vi "Core_Chem_User_Interface_v1.4.vi"() -> ()   [LabVIEW 2014]
uses:
  <vilib>/dex/Stream Element Allocation Mode.ctl
  C:/Program Files (x86)/National Instruments/LabVIEW 2014/examples/Data Communication/Network Streams/Simple Network Streams/support/Network Stream Command.ctl
  <vilib>/Platform/TimedLoop/XDataNode/timing_clust.ctl
  <vilib>/Platform/TimedLoop/XDataNode/nitl_modes.ctl
  <vilib>/Platform/TimedLoop/XDataNode/wakeup.ctl
  <vilib>/Utility/tcp.llb/UDP Multicast Read-Only Open.vi
  <vilib>/platform/TimedLoop/XDataNode/XDataNode.xnode
  <vilib>/Platform/TimedLoop/XDataNode/XDNodeRunTimeDep.lvlib
  <vilib>/FTP/NI_FTP.lvlib
panel:
  out "Create folder error out 2":errorcluster
  out "Network to cRIO live status":bool
  out "Create folder error out":errorcluster
  in  "Confirm Flight Number":bool
  out "PRTAFT_UDP_In":string
  out "TWBOZO01":string
  out "CABOZO01":string
  out "TEIOZO01":string
  out "CHTSOO01":string
  out "CHFGGA01":string
  out "AL52CO01":string
  in  "Flight Number":string
  in  "Tab Control":T1(tab)
  out "FGGA preflight Des 17":string="Preflight - Start minimum 2 hours before take-off\n\n1. Ensure no bags/jackets are stowed on seat backs and behind seats in front of core chemistry rack at all times.\n\n2. Remove inlet covers if applicable.\n\n3. Connect Lilliput mini TFT/LCD VGA cable to FGGA VIDEO (back panel) and PS2 Keyboard/Mouse cables to FGGA Connectors (back panel). TFT/LCD and Keyboard kept in Core Chemistry Dell laptop bag. Connect TFT/LCD AC/DC PSU to 6026-8-98 Amphenol (SSP9) and make 230 Vac CB.\n\n4. Ensure all circuit breakers are pushed in, except 230Vac and 28Vdc, UPS switch off (down) and AL5002 CO Plasma Lamp switch off (down), WoW key to normal (horizontal).\n\n5. Wait for ALL network swtiches on the aircraft to be up and running before start-up.\n\n6. Check AboutTime has synchronised laptop clock to aircraft timeservers (Filiberto/Gaston).\n\nClick the PowerUp Tab."
  out "FGGA preflight Des 16":string="PowerUp\n\n1.\tSSP9 forward face\tMake 3 CBs\n\n2.\tPWRDIST \t\tMake 230Vac CB \n                     Switch UPS On \t[UP]\n                     Make 28Vdc CB\n                     Check 28VDC OK Green Light comes on\n\n3.\tCore Chemistry e-Log\nComplete Core Chemistry e-Log in WordPad (Bnnn_CoreChemLog_v2.2), save on Flight Manager's laptop (192.168.101.180/      flt_folders/Bnnn); Fill in header with date, flight number and your name/initials.\n\n4.\tSAMPUMP\t\t\n - Switch WoW override key (vertical) to check pump starts, and MFM flowrate increase (>20 LPM) on the right hand plot. \n - Switch off WoW override\t\t\t\t [NORM, key horizontal]\n\nClick the 2B Ozone tab if operated, otherwise, click the UDP tab.\n\n\n"
  out "MFM":dbl(graph)
  in  "Ambient = OFF\nCabin = ON":bool
  out "FGGA preflight Des 15":string="2B Ozone Preflight\n\n1.\tSelect either Ambient or Cabin Air mode (default should be OFF for Ambient air mode).\n\n2. Check flowrate is greater than 2000 sccm on the right hand plot.\n\nClick the UDP tab."
  out "2B Ozone concentration":dbl(graph)
  out "2B Ozone flow rate":dbl(graph)
  out "2BOzone Event error out":errorcluster
  out "2BOzone command sender error out":errorcluster
  out "FGGA preflight Des 20":string="4. Check derived parameters in DECADES (192.168.101.110 & 192.168.101.108). 574 Ozone TEi49C; 588 CO AL5002; 611 SO2 TEi43i; 903 - 905 FGGA; 910 / 920 Ozone 2B."
  out "FGGA preflight Des 14":string="UDP Preflight\n1. Check all UDP packets are updating.  Unix time increasing by 1 sec (3rd parameter).\n2. Check flight number is correct.\n3. Confirm flight number and check it appears in the UDP packet (6th parameter). "
  in  "name":string="239.1.4.6"
  in  "Port":u16=50001
  out "FGGA":string
  out "CO":string
  out "Ozone":string
  out "Cabin Ozone":string
  out "Ambient Ozone":string
  out "SO2":string
  out "Ozone Zeroing\nTime Remain (sec)":u32
  in  "Ozone Zeroing":bool
  out "TEI49C Sample Flow B":dbl(graph)
  out "TEi49C Concentration":dbl(graph)
  out "TEI49C Sample Flow A":dbl(graph)
  out "FGGA preflight Des 13":string="TEi49C Ozone PRE-FLIGHT - LAST ACTIONS BEFORE SEAT-BELTING DOWN (PRIOR TO ENGINES START)\n\n1. Ozone monitor zeroing\t\t[10 min minimum]\n\n\n2. Check TEi49C zero value and note down value in e-Log. \n"
  out "FGGA preflight Des 12":string="TEi49C Ozone Preflight\n\n1. Check nominal sample flowrate on both channels is ~0.7 LPM."
  out "Ozone Event error out":errorcluster
  out "Ozone command sender error out":errorcluster
  in  "Ozone UDP Time Offset":i32=1
  in  "eV9 Flush User\nset time (sec)":i32=15
  in  "MFC_3 User Set Value":dbl=2.0
  in  "MFC_2 User Set Value":dbl=2.5
  out "SO2 Zeroing (Inflight)\nTime Remain (sec)":u32
  in  "eV6 User set time \n(Inflight) (sec)":i32=120
  in  "eV6 User\nset time (sec)":i32=600
  in  "SO2 Inflight \nZeroing":bool
  out "SO2 Flush\nTime Remain (sec)":u32
  out "TEI43i MFC3 Sample Flow":dbl(graph)
  out "TEi43C / TEi43i Concentration":dbl(graph)
  out "TEI43C Sample Flow":dbl(graph)
  out "TEI43i MFC2 Cal Flow":dbl(graph)
  out "SO2 CAL\nTime Remain (sec)":u32
  out "SO2 Cal Flush\nTime Remain (sec)":u32
  in  "SO2 CAL":bool
  out "FGGA preflight Des 11":string="TEi43 SO2 Inflight Calibration & Zeroing"
  in  "SO2 Zeroing":bool
  out "SO2 Zeroing\nTime Remain (sec)":u32
  out "FGGA preflight Des 10":string="TEi43 SO2 PRE-FLIGHT - LAST ACTIONS BEFORE SEAT-BELTING DOWN (PRIOR TO ENGINES START)\n\n1. SO2 monitors zeroing\t\t[10 min minimum]\n\n\n2. Check TEi43i or TEi43C zero value and note down value in e-Log. "
  in  "SO2 Flush":bool
  out "FGGA preflight Des 9":string="TEi43 SO2 Preflight\n\n1. Check nominal sample flowrate is 2.0 LPM on the right hand plot.\n\nSO2 calibration gas purge - SO2 calibration cylinder locate at bottom of WAS Gas rack.\n\n2. Check quick connect male body is connected to 'chem 1' gas line.\n\n3. Open cylinder valve 1.\n\n4. Set regulator (V2) to deliver at 3 bar.\n\n5. Open regulator valve 3 (anti-clockwise).\n\n6. Close cylinder valve 1.\n\n\n7. Press SO2 flush button, MFC2 cal flow should increase to 2.5 SLPM.\nMonitor MFC2 flow rate to make sure the reading decreases from 2.5 SLPM to 0.0 SLPM.\nCheck pressure content and delivery gauges also reads zero.\nIf pressure content & delivery gauges do NOT read zero, press SO2 flush button again until they do.\n\n8. Quickly open and close cylinder valve 1.\n\n9. Repeat step 7) to 8) three times.\n\n10. Open cylinder valve 1, system is ready. Note down content pressure in elog.\n "
  in  "eV9 flush User\nset time (sec)":i32=60
  in  "eV8 User\nset time (sec)":i32=120
  out "SO2 Event error out":errorcluster
  out "SO2 command sender \nerror out":errorcluster
  in  "SO2 UDP Time Offset":i32=1
  out "Lamp Temperature":dbl(graph)
  out "CO CAL Status":bool
  in  "CO CAL":bool
  out "FGGA preflight Des 8":string="CO Preflight and Inflight Calibrations\nHold down the CAL button for 2 secs then release, CAL status should then lit up.\nInflight calibration performed on 45 minutes interval or more frequently if lamp temperature > 35.5 degC."
  in  "Prepare Gases":bool
  out "FGGA preflight Des 7":string="AL5002 CO Preflight Checks\n\n1.\n\n2. Start CO Vacuum. NB: If there is problem with the software control, use manual override switch [up] on CALDECK front panel\n\n3. CO Checks - charts on the right hand side\n    Lamp Flow Controller ~ 40 ml/min\n    Monochromator Flow Controller ~ 30 ml/min\n    Fluorescence Cell Pressure ~ 7.5 Torr\n\nIf Lamp/Mono flows are low, manual valves (V1 -> V5) may still be shut, or pressure adjusting valves (ALREG1 & 2) have not been set > 2 bar\n\nIf Cell pressure is 10 Torr (max range), check that COPUMP is running and eV7 is opened (CO Vacuum eV7 is ON).\n\n4. Switch Plasma Lamp at the front panel UP\n\nDetector count rate (on 'Raw Signal' or F2 instrument touchscreen) should increase to >=10000 Hz within a minute.  Recycle plasma lamp switch (off/on) if no significant increase in count rate after 10 mins.  CO concentration should increase (100s ppb). \n     \n\n"
  in  "CO Vaccum (eV7)":bool
  out "Raw Signal":dbl(graph)
  out "CO Concentration":dbl(graph)
  out "Fluorescence Cell Pressure":dbl(graph)
  out "Monochromator Flow":dbl(graph)
  out "Lamp Flow Controller":dbl(graph)
  in  "CO UDP Time Offset":i32=1
  out "CO2 Pressure\nDelivery (PSIA)":dbl(slide) scale=0.0..100.0
  out "Std\nContent (barG)":dbl(slide) scale=0.0..220.0
  out "N2\nContent (barG)":dbl(slide) scale=0.0..220.0
  out "CO2\nContent (barG)":dbl(slide) scale=0.0..170.0
  out "CO Event error out":errorcluster
  out "CO command sender error out":errorcluster
  out "CO Zero":T2(array[cluster])
  out "CO Sensitivity":T3(array[cluster])
  out "Ring Down Time RDA & RDB":cluster{dbl, dbl}(graph)
  in  "Line Lock Setting Change":bool
  out "Cell temperature":dbl(graph)
  out "Cell pressure":dbl(graph)
  in  "Manual FGGA Pump":bool
  out "CO2":dbl(graph)
  out "CH4":dbl(graph)
  out "H2O":dbl(graph)
  out "WoW Flag":string="0"
  in  "FGGA pump\nsync to WoW":bool
  out "CH4 Dry":dbl(graph)
  out "CO2 Dry":dbl(graph)
  out "MFC1 Cal Flow":dbl(graph)
  out "Flush Target Tank\nTime Remain (sec)":u32
  out "Flush Low Tank\nTime Remain (sec)":u32
  out "Flush High Tank\nTime Remain (sec)":u32
  in  "Flush Target Tank":bool
  in  "Flush Low Tank":bool
  in  "Flush High Tank":bool
  in  "FGGA Restart":bool
  out "FGGA preflight Des 6":string="FGGA Instrument Controls"
  in  "High Cal":bool
  out "High Cal\nFlush Time Remain (sec)":u32
  out "High Cal\nCal Time Remain (sec)":u32
  in  "Low Cal":bool
  in  "Target Cal":bool
  in  "Span Cal - \nHigh Cal, CO Cal, Low Cal":bool
  out "Low Cal\nFlush Time Remain (sec)":u32
  out "Low Cal\nCal Time Remain (sec)":u32
  out "Target Cal\nFlush Time Remain (sec)":u32
  out "Target Cal\nCal Time Remain (sec)":u32
  in  "MFC_1 User Set Value":dbl=2.0
  out "FGGA preflight Des 5":string="FGGA Inflight Calibrations"
  out "FGGA preflight Des 4":string="FGGA Ground Preflight Checks\n\n1. Switch FGGA pump ON\n\n2. Check cavity pressure ~50 Torr\n\n3. Switch FGGA pump OFF\n\n4. Enable FGGA pump sync to WoW\n\n5.. Check Time Synchronisation\n\n6. Check CO2 & CH4 values\n\nIf CO2 & CH4 values are -1 ppm, follow the \nchange linelock settings procedure.\n\n\n\n\n\nLAST ACTION BEFORE SEAT-BELTING \nDOWN (PRIOR TO ENGINES START)\n\n1. Disconnect Monitor & stow away. Leave Keyboard & Mouse connected. Place keyboard at the bottom\nof the rack.\n\n"
  out "FGGA preflight Des 3":string="FGGA CAL Gas Purge\n\nFor each cylinder in gas stowage, check that,\n\n1. V1 Closed\n    V3 Closed\n    V4 Make sure arrow positioned downwards (i.e. flow points to gas line)\n\n2. V3 Open (turn anti-clockwise)\n\n3. Use the button on the right according to the operating cylinder to flush the line. Monitor the MFC flow rate to make sure the reading decreases from 3 to zero. (ie fully flushed). Pressure content & delivery gauges should also read zero.\n\n4. V3 Close (turn clockwise)\n\n5. V1 Open / Close quickly\n         Check delivery pressure gauge is ~ 40 PSI \n         (Use V2 to increase if necessary)\n\n6. Repeat steps 2) to 5) three times\n\n7. V3 Close (turn clockwise)\n\n8. V1 Open, check V2 ~ 40 PSIG\n\n9. V3 Open - System is ready"
  out "FGGA command sender error out":errorcluster
  out "FGGA Event Error out":errorcluster
  in  "FGGA UDP Time Offset":i32=1
  in  "FGGA Shutdown":bool
  in  "Postflight Procedures":bool
  in  "cRIO File IO Stop\n(USB Flash Drive Unmount)":bool
  in  "FTP ASCII Files to Local":bool
  in  "Transfer FGGA Files":bool
  out "FGGA preflight Des 18":string="Postflight\n\n1. Press the cRIO File IO Stop to stop ASCII file recording\nNote: ASCII file recording will start again once a new  flight number is confirmed.\n\n2. Press the FTP ASCII File to Local button to transfer ASCII files to flight folder.\n\n\n3. Press the Transfer FGGA Files button to transfer FGGA files to flight folder. \n\n4. Shutdown FGGA.\n\n\n5. View Postflight Procedures."
  out "File List":string[](array[string])
  out "FGGA File Transfer Error out":errorcluster
  out "Move to FM Error out":errorcluster
  out "USB Disk Space Used %":dbl(slide) scale=0.0..100.0
  out "PTP Sync":bool
  out "CPU Total %":dbl(graph)
  out "PRTAFT_DLU":string
  out "FGGA preflight Des 19":string="This tab controls ONLY for advanced operators."
  in  "Inst_alm_thresh":i32=220
  in  "3hr_alm_thresh":i32=80
  in  "Simulate Inst Conc":i32
  in  "Simulate 3hr Average Conc":dbl
  in  "Simulate 2B Conc":bool
  in  "Ozone eV6":bool
  in  "Simulate Conc":bool
  in  "8hr TWA Limit":i32=490
  in  "10mins STEL Limit":i32=700
  in  "SO2 Slope":dbl=1.0
  in  "SO2 Offset":dbl
  in  "Simulate TWA Conc":dbl
  in  "Simulate STEL Conc":dbl
  in  "MFC_3\nSLPM Value":dbl=2.0
  in  "MFC_2\nSLPM Value":dbl
  in  "SO2 eV6":bool
  in  "eV8":bool
  in  "eV9":bool
  in  "eV4":bool
  in  "eV3":bool
  in  "MFC_1\nSLPM Value":dbl
  in  "eV2":bool
  in  "eV1":bool
  # "Unix time"
  # "Flight Number"
  # "Unix time"
  # "Unix time"
  # "Unix time"
  # "Unix time"
  # "concentration\npmt_volt\nlamp_volt\nlamp_intens\ninternal_temper\nreact_temper\nreact_press\nflow\nflags\nten_min_so2\neight_hr_so2\nten_min_so2_alm\neight_hr_so2_alm\nMFC_2absolute_pres\nMFC_2temperature\nMFC_2volumetic_flow\nMFC_2mass_flow\nMFC_2set_point\nMFC_3_absolute_pres\nMFC_3_temperature\nMFC_3volumetic_flow\nMFC_3mass_flow\nMFC_3set_point\nV6\nV8\nV9\nMFC2_Set_Value\nMFC3_Set_Value"
  # "Flight Number"
  # "Flight Number"
  # "Flight Number"
  # "Flight Number"
  # "conc\ntemp\npress\nflow\nthreehr_oz\nInst_alarm\nthreehr_alarm"
  # "ch4\nco2\nh2o\npress_torr\ntemp_c\nfit_flag\nrda_usec\nrdb_usec\nch4_dry\nco2_dry\nMFC_1_absolute_pres\nMFC_1_temperature\nMFC_1volumetic_flow\nMFC_1mass_flow\nMFC_1set_point\nV1\nV2\nV3\nV4\nrestart_FGGA\nFGGA_Pump\nCAL_MFC_1Set_Value"
  # "conc\ntemp\npress\nflow"
  # "conc\nbenchtemp\npress\ncellAint\ncellBint\nFlowA\nFlowB\nlamptemp\nflag\nV6"
  # "conc\ncounts\nsens\nzero\nlampflow\nlamptemp\nmonoflow\nmonotemp\nmonopress\ncellpress\ncalpress\ntemppmt\ncalconc\nerr\ncal_counter\nerr_counter\nCO_vacuum_status\nIn_Cal\nALEG1_press_delivery\nALREG1_press_content\nALREG2_press_content\nALREG3_press_content"
  # "TEi43c"
  # "TEi43i"
  # "V3"
  # "V2"
  # "V1"
  # "SO2 CAL SETTINGS"
  # "FGGA"
  # "2B Ozone"
  # "TEi49C  - Ozone"
  # "TEi43 - SO2"
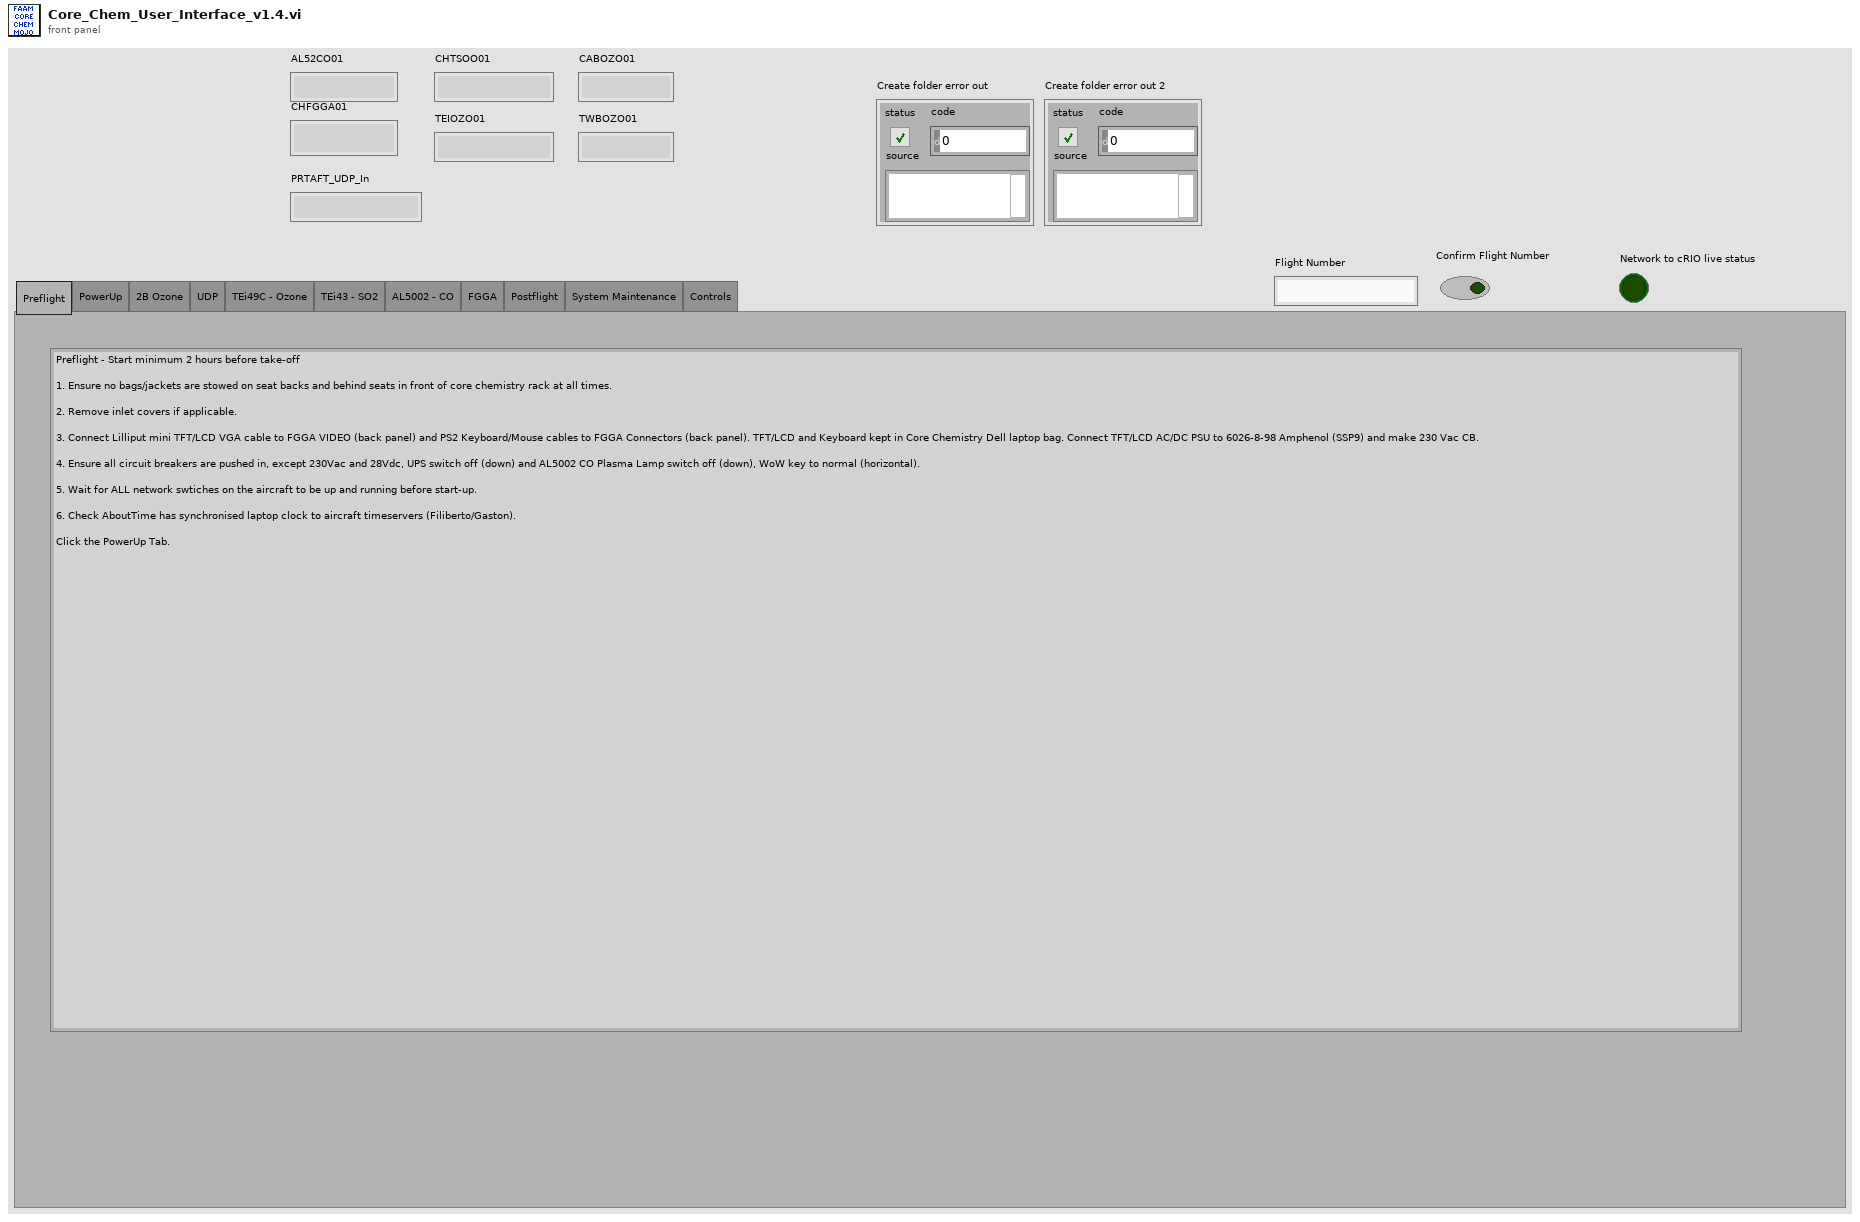
[diagram p1: front panel]
types:
  T1 = enum32{"Preflight", "PowerUp", "2B Ozone", "UDP", "TEi49C - Ozone", "TEi43 - SO2", "AL5002 - CO", "FGGA", "Postflight", "System Maintenance", "Controls"}
  T2 = cluster{"time stamp":timestamp, "CO Offset":dbl}[]
  T3 = cluster{"time stamp":timestamp, "CO Sensitivity":dbl}[]
  T4 = typedef "Network Stream Command.ctl" = cluster{"Message":string, "Message Data":variant}
  T5 = typedef "Stream Element Allocation Mode.ctl" = u32
  T6 = typedef "XDNodeRunTimeDep.lvlib/timing_clust.ctl" = cluster{"Expected End [f-1]":u64, "Actual End [f-1]":u64, "Finished Late? [f-1]":bool, "Expected End [i-1]":u64, "Actual End [i-1]":u64, "Finished Late? [i-1]":bool, "Expected Start [i]":u64, "Actual Start [i]":u64, "Expected Start [f]":u64, "Actual Start [f]":u64, "Source Name":string, "Structure Name":string, "Period":i64, "Deadline":i64, "Offset":i64, "Start":i64, "Priority":i32, "Timeout":i32, "Mode":T7, "Wakeup Reason":T8, "Error":errorcluster, "Source Type":string, "Secondary Source Type":string, "Global End Time":u64, "Global Start Time":u64, "Frame Duration":u64, "Iteration Duration":u64, "Assigned CPU":i32, "I/O Scan Engine Mode":u32}
  T7 = typedef "XDNodeRunTimeDep.lvlib/nitl_modes.ctl" = enum32{"No Change", "Process missed periods, maintain original phase", "Discard missed periods, maintain original phase", "Process missed periods, ignore original phase", "Discard missed periods, ignore original phase"}
  T8 = typedef "XDNodeRunTimeDep.lvlib/wakeup.ctl" = enum32{"Normal", "Aborted", "Asynchronous wakeup", "Timing source error", "Timed loop error", "Timeout"}
  T9 = typedef "NI_FTP.lvlib/FTP Session.ctl" = refnum<k5>
  T10 = typedef "NI_FTP.lvlib/FTP File Info.ctl" = cluster{"type":enum16{"unknown", "file", "dir", "link"}, "permissions":string, "owner":string, "group":string, "size":i32, "date":string, "name":string, "link name":string}
  T11 = cluster{"Message":string, "Message 2":string, "Message 3":string}
  T12 = cluster{"Message":string, "Message 2":string, "Message 3":string, "Message 4":string}
  T13 = cluster{"Message":string, "Message 3":string, "Message 4":string}
diagram:
  w4 = "XXXX"
  w7 = 0
  w8 = 0.0
  w14 = T4 {"Message"="", "Message Data"=variant} ("Message Cluster")
  w20 = T5 0 items=["allocate as needed", "pre-allocate"] ("element allocation mode")
  w26 = T4 {"Message"="", "Message Data"=variant} ("Message Cluster")
  w32 = T5 0 items=["allocate as needed", "pre-allocate"] ("element allocation mode")
  w37 = T4 {"Message"="", "Message Data"=variant} ("Message Cluster")
  w43 = T5 0 items=["allocate as needed", "pre-allocate"] ("element allocation mode")
  w53 = T5 0 items=["allocate as needed", "pre-allocate"] ("element allocation mode")
  w55 = T4 {"Message"="", "Message Data"=variant} ("Message Cluster")
  w62 = T5 0 items=["allocate as needed", "pre-allocate"] ("element allocation mode")
  w64 = T4 {"Message"="", "Message Data"=variant} ("Message Cluster")
  n1 = local write "cRIO File IO Stop\n(USB Flash Drive Unmount)"(FALSE ("Stop File Write")) -> ()
  n2 = local write "Flight Number"(w4) -> ()
  n3 = while {
    shift-right: [w68] -> _
    shift-left: w4 -> [w67]
    stop <- FALSE stop-if-true
    n4 = Not Equal?(x=w67, y="Flight Number") -> (x != y?=w70:bool)
    n5 = case shown="True" w70 {
      tunnel: [w73 w74] -> w68
      tunnel: "Flight Number" -> [_ w74]
      tunnel: w67 -> [w73 _]
      frame False {
      }
      frame True {
        n6 = One Button Dialog(message="Flight Number changed,\nPress flight number button to confirm") -> ()  [unwired: 1 in, 1 out]
      }
    }
    n7 = Wait (ms)(milliseconds to wait=u32 1000) -> ()  [unwired: 1 out]
  }
  n8 = while {
    stop <- FALSE stop-if-true
    # "UDP Read"
    n9 = String To IP(1:"name") -> (0:w81:u32)
    n10 = call-poly <vilib>:"UDP Multicast Open.vi"("multicast addr"=w81, "port"="Port") -> ("error out"=w79:errorcluster, "connection ID"=w78:refnum<k16>)  [unwired: 7 in, 1 out]
    n11 = Wait (ms)(milliseconds to wait=u32 1000) -> ()  [unwired: 1 out]
    n12 = case shown="No Error" w79 {
      selector: w79 -> [w85 _]
      tunnel: w78 -> [w84 _]
      frame No Error {
        w83 = ""
        n13 = while {
          tunnel: w85 -> [w131]
          tunnel: w84 -> [w130]
          shift-right: [w126] -> _
          shift-left: w83 -> [w127]
          shift-right: [w117] -> _
          shift-left: w83 -> [w119]
          shift-right: [w111] -> _
          shift-left: w83 -> [w113]
          shift-right: [w105] -> _
          shift-left: w83 -> [w106]
          shift-right: [w99] -> _
          shift-left: w83 -> [w100]
          shift-right: [w93] -> _
          shift-left: w83 -> [w94]
          shift-right: [w87] -> _
          shift-left: w83 -> [w88]
          stop <- w129 stop-if-true
          n14 = UDP Read(connection ID=w130, 8:w131) -> (data out=w86:string, error out=w129:errorcluster)  [unwired: 2 in, 3 out]
          n15 = Match Pattern(string=w86, regular expression="$TEIOZO01,") -> (match substring=w125:string, after substring=w124:string)  [unwired: 1 in, 2 out]
          n16 = Match Pattern(string=w86, regular expression="$TWBOZO01,") -> (match substring=w103:string, after substring=w102:string)  [unwired: 1 in, 2 out]
          n17 = Match Pattern(string=w86, regular expression="$CABOZO01,") -> (match substring=w109:string, after substring=w108:string)  [unwired: 1 in, 2 out]
          n18 = Match Pattern(string=w86, regular expression="$CHTSOO01,") -> (match substring=w97:string, after substring=w96:string)  [unwired: 1 in, 2 out]
          n19 = Match Pattern(string=w86, regular expression="$CHFGGA01,") -> (match substring=w121:string, after substring=w120:string)  [unwired: 1 in, 2 out]
          n20 = Match Pattern(string=w86, regular expression="$AL52CO01,") -> (match substring=w115:string, after substring=w114:string)  [unwired: 1 in, 2 out]
          n21 = Match Pattern(string=w86, regular expression="$PRTAFT01,") -> (match substring=w92:string, after substring=w91:string)  [unwired: 1 in, 2 out]
          n22 = Concatenate Strings(w125, w124) -> (w123:string)
          n23 = Concatenate Strings(w103, w102) -> (w101:string)
          n24 = Concatenate Strings(w109, w108) -> (w107:string)
          n25 = Concatenate Strings(w97, w96) -> (w95:string)
          n26 = Concatenate Strings(w121, w120) -> (w118:string)
          n27 = Concatenate Strings(w115, w114) -> (w112:string)
          n28 = Concatenate Strings(w92, w91) -> (w89:string)
          n29 = Replace Substring(4:w101, 5:w100) -> (1:w99:string)  [unwired: 2 in, 1 out]
          "TWBOZO01" <- w99
          n30 = Replace Substring(4:w123, 5:w127) -> (1:w126:string)  [unwired: 2 in, 1 out]
          "TEIOZO01" <- w126
          n31 = Replace Substring(4:w107, 5:w106) -> (1:w105:string)  [unwired: 2 in, 1 out]
          "CABOZO01" <- w105
          n32 = Replace Substring(4:w95, 5:w94) -> (1:w93:string)  [unwired: 2 in, 1 out]
          "CHTSOO01" <- w93
          n33 = Replace Substring(4:w112, 5:w113) -> (1:w111:string)  [unwired: 2 in, 1 out]
          "AL52CO01" <- w111
          n34 = Replace Substring(4:w118, 5:w119) -> (1:w117:string)  [unwired: 2 in, 1 out]
          "CHFGGA01" <- w117
          n35 = Replace Substring(4:w89, 5:w88) -> (1:w87:string)  [unwired: 2 in, 1 out]
          "PRTAFT_UDP_In" <- w87
        }
      }
      frame Error {
      }
    }
  }
  n36 = Obtain Queue(name (unnamed)="CO_Command", element data type=w64) -> (queue out=w13:refnum<queue>, error out=w58:errorcluster)  [unwired: 3 in, 1 out]
  n37 = Create Network Stream Writer Endpoint(6:w62, 7:10 ("writer buffer size"), 9:w64, 10:"//192.168.101.17/command/reader/CO" ("reader url"), 11:"/command/writer/CO" ("writer name")) -> (0:w61:errorcluster, 3:w60:refnum<k21>)  [unwired: 2 in]
  n38 = while {
    tunnel: w13 -> [w135]
    tunnel: w58 -> [w134]
    tunnel: [w132] -> _
    stop <- FALSE stop-if-true
    # "CO UI Event Handler Loop"
    n39 = event shown="[4] \"Confirm Flight Number\": Value Change" {
      selector: _ -> [_ _ _ _ _]
      dyn-events: _ -> [_ _ _ _ _]
      timeout: _ -> [_ _ _ _ _]
      tunnel: w135 -> [w142 w149 w153 w160 w168]
      tunnel: w134 -> [w141 w148 w152 w159 w167]
      tunnel: [w136 w143 w151 w158 w166] -> w132
      event "CO CAL": Value Change {
        n40 = event-data() -> ("NewVal"=w139:bool)  [unwired: 1 in]
        n41 = Bundle(cluster=T4 {"Message"="", "Message Data"=variant} ("Message Cluster"), "Message"="CO CAL", "Message Data"=w139) -> (w137:T4)
        n42 = Enqueue Element(queue=w142, element=w137, error in (no error)=w141) -> (error out=w136:errorcluster)  [unwired: 1 in, 2 out]
      }
      event "CO UDP Time Offset": Value Change {
        n43 = event-data() -> ("NewVal"=w146:i32)  [unwired: 1 in]
        n44 = Bundle(cluster=T4 {"Message"="", "Message Data"=variant} ("Message Cluster"), "Message"="UDP Time Offset", "Message Data"=w146) -> (w144:T4)
        n45 = Enqueue Element(queue=w149, element=w144, error in (no error)=w148) -> (error out=w143:errorcluster)  [unwired: 1 in, 2 out]
      }
      event "CO Vaccum (eV7)": Value Change {
        n46 = event-data() -> ("NewVal"=w150:bool)  [unwired: 1 in]
        n47 = Bundle(cluster=T4 {"Message"="", "Message Data"=variant} ("Message Cluster"), "Message"="CO Vacuum", "Message Data"=w150) -> (w154:T4)
        n48 = Enqueue Element(queue=w153, element=w154, error in (no error)=w152) -> (error out=w151:errorcluster)  [unwired: 1 in, 2 out]
      }
      event "cRIO File IO Stop\n(USB Flash Drive Unmount)": Value Change {
        n49 = event-data() -> ("NewVal"=w157:bool)  [unwired: 1 in]
        n50 = Bundle(cluster=T4 {"Message"="", "Message Data"=variant} ("Message Cluster"), "Message"="Stop File Write", "Message Data"=w157) -> (w161:T4)
        n51 = Enqueue Element(queue=w160, element=w161, error in (no error)=w159) -> (error out=w158:errorcluster)  [unwired: 1 in, 2 out]
      }
      event "Confirm Flight Number": Value Change {
        n52 = event-data() -> ()  [unwired: 1 in, 1 out]
        n53 = flat-sequence {
          tunnel: w167 -> [w170]
          tunnel: w168 -> [w171]
          tunnel: [w171] -> w165
          tunnel: [w170] -> w164
          tunnel: [w173] -> w166
          tunnel: w165 -> [w175]
          tunnel: w164 -> [w174]
          frame #0 {
            n54 = local write "cRIO File IO Stop\n(USB Flash Drive Unmount)"(FALSE ("cRIO File IO Stop\n(USB Flash Drive Unmount)")) -> ()
          }
          frame #1 {
            n55 = local read "Flight Number"() -> (w172:string)
            n56 = Bundle(cluster=T4 {"Message"="", "Message Data"=variant} ("Message Cluster"), "Message"="Flight Number", "Message Data"=w172) -> (w176:T4)
            n57 = Enqueue Element(queue=w175, element=w176, error in (no error)=w174) -> (error out=w173:errorcluster)  [unwired: 1 in, 2 out]
          }
        }
      }
    }
    "CO Event error out" <- w132
  }
  n58 = while {
    tunnel: w13 -> [w186]
    shift-right: [w181] -> _
    shift-left: w60 -> [w183]
    shift-right: [w179] -> w49
    shift-left: w61 -> [w185]
    tunnel: w58 -> [w180]
    stop <- w179 stop-if-true
    # "CO UI Command Sender"
    n59 = Dequeue Element(queue=w186, error in (no error)=w180) -> (element=w182:T4)  [unwired: 1 in, 3 out]
    n60 = Unbundle By Name(w182) -> ("Message"=w184:string)
    n61 = case shown="\"UDP Time Offset\"" w184 {
      tunnel: w185 -> [w187 w191 w198 w205 w212 w219]
      tunnel: w183 -> [w188 w194 w201 w208 w215 w222]
      tunnel: w182 -> [_ w193 w200 w207 w214 w221]
      tunnel: [w187 w190 w197 w204 w211 w218] -> w179
      tunnel: [w188 w189 w196 w203 w210 w217] -> w181
      frame "False", Default {
      }
      frame "CO CAL" {
        n62 = shared-variable-write(w194, w191, w193) -> (w192:refnum<k21>, w195:errorcluster)  [unwired: 1 in, 1 out]
        n63 = Flush Stream(8:w195, 11:w192) -> (0:w190:errorcluster, 3:w189:refnum<k21>)  [unwired: 2 in, 1 out]
      }
      frame "UDP Time Offset" {
        n64 = shared-variable-write(w201, w198, w200) -> (w199:refnum<k21>, w202:errorcluster)  [unwired: 1 in, 1 out]
        n65 = Flush Stream(8:w202, 11:w199) -> (0:w197:errorcluster, 3:w196:refnum<k21>)  [unwired: 2 in, 1 out]
      }
      frame "Stop File Write" {
        n66 = shared-variable-write(w208, w205, w207) -> (w206:refnum<k21>, w209:errorcluster)  [unwired: 1 in, 1 out]
        n67 = Flush Stream(8:w209, 11:w206) -> (0:w204:errorcluster, 3:w203:refnum<k21>)  [unwired: 2 in, 1 out]
      }
      frame "Flight Number" {
        n68 = shared-variable-write(w215, w212, w214) -> (w213:refnum<k21>, w216:errorcluster)  [unwired: 1 in, 1 out]
        n69 = Flush Stream(8:w216, 11:w213) -> (0:w211:errorcluster, 3:w210:refnum<k21>)  [unwired: 2 in, 1 out]
      }
      frame "CO Vacuum" {
        n70 = shared-variable-write(w222, w219, w221) -> (w220:refnum<k21>, w223:errorcluster)  [unwired: 1 in, 1 out]
        n71 = Flush Stream(8:w223, 11:w220) -> (0:w218:errorcluster, 3:w217:refnum<k21>)  [unwired: 2 in, 1 out]
      }
    }
  }
  "CO command sender error out" <- w49
  n72 = node-c288() -> (w12:T6)  [unwired: 4 in]
  n73 = Initialize Array(cluster{"time stamp":timestamp, "Y":dbl} {"time stamp"=timestamp(0 s since 1904-01-01), "Y"=0.0}, 30 ("dimension size")) -> (w9:cluster{"time stamp":timestamp, "Y":dbl}[])
  n74 = timed-loop {
    timing: w12 -> [_]
    timing-out: [_] -> w11
    stop <- _ stop-if-true
    # "PC Tasks"
    n75 = node-c288() -> ()  [unwired: 1 in, 1 out]
    n76 = event shown="[0] \"FTP ASCII Files to Local\": Value Change" {
      selector: _ -> [_ _ _ _]
      dyn-events: _ -> [_ _ _ _]
      timeout: _ -> [_ _ _ _]
      event "FTP ASCII Files to Local": Value Change {
        n77 = event-data() -> ()  [unwired: 1 in, 1 out]
        n78 = flat-sequence {
          tunnel: [w232] -> w226
          tunnel: [w244] -> w231
          tunnel: [w243] -> w229
          tunnel: [w242] -> w227
          tunnel: w226 -> [w242]
          tunnel: w231 -> [w302]
          tunnel: [w302] -> w230
          tunnel: w229 -> [w298]
          tunnel: [w297] -> w228
          tunnel: w227 -> [w297]
          tunnel: w230 -> [w308]
          tunnel: w228 -> [w303]
          frame #0 {
            n79 = local read "Flight Number"() -> (w234:string)
            n80 = Concatenate Strings("Confirm Flight Number" ("message"), "\n", w234) -> (w238:string)
            n81 = Two Button Dialog(message=w238, 1:"No" ("F button name (\"Cancel\")"), 2:"Yes" ("T button name (\"OK\")")) -> (T button?=w235:bool)
            n82 = case shown="False" w235 {
              tunnel: w234 -> [_ w241]
              tunnel: [w240 w241] -> w232
              frame False {
                n83 = call "Prompt User for Flight Number2"() -> ("Flight Number BXXX"=w240:string)  [unwired: 17 in, 2 out]
              }
              frame True {
              }
            }
          }
          frame #1 {
            n84 = Get Date/Time In Seconds() -> (seconds since 1Jan1904=w248:timestamp)
            n85 = Format Date/Time String(time format string (%c)="%Y%m%d", seconds (now)=w248) -> (date/time string=w246:string)  [unwired: 1 in]
            n86 = call <vilib>:"FTP Open Session.vi"("address"="192.168.101.17") -> ("error out"=w263:errorcluster, "ftp session"=w264:T9)  [unwired: 7 in, 2 out]
            n87 = Concatenate Strings("Use Today's Date" ("message"), "\r", w246) -> (w252:string)
            n88 = call <vilib>:"FTP Logon.vi"("error in (no error)"=w263, "password"="", "user"="anonymous", "ftp session"=w264) -> ("error out"=w260:errorcluster, "ftp session out"=w259:T9)  [unwired: 4 in, 2 out]
            n89 = Two Button Dialog(message=w252, 1:"No" ("F button name (\"Cancel\")"), 2:"Yes" ("T button name (\"OK\")")) -> (T button?=w249:bool)
            n90 = case shown="False" w249 {
              tunnel: [w267 w268] -> w243
              tunnel: w246 -> [_ w268]
              frame False {
                n91 = call "Prompt User for Date"() -> ("Date"=w267:string)  [unwired: 17 in, 2 out]
              }
              frame True {
              }
            }
            n92 = call <vilib>:"FTP Directory Listing.vi"("error in (no error)"=w260, "directory path"="/U:/data", "ftp session"=w259) -> ("dir list"=w258:T10[])  [unwired: 4 in, 4 out]
            n93 = for {
              tunnel: w258 -> [w288] mode=indexing
              tunnel: [w287] -> w255 mode=indexing
              tunnel: w243 -> [w286]
              # "Extract File Name According to the Date"
              n94 = Unbundle By Name(w288) -> ("name"=w294:string, "name"=w293:string)
              n95 = Match Pattern(string=w293, regular expression="_[0-9]+") -> (match substring=w291:string)  [unwired: 1 in, 3 out]
              n96 = String Subset(string=w291, offset (0)=1) -> (substring=w289:string)  [unwired: 1 in]
              n97 = Equal?(x=w289, y=w286) -> (x = y?=w295:bool)
              n98 = case shown="False" w295 {
                tunnel: w294 -> [_ w296]
                tunnel: [_ w296] -> w287
                frame False {
                }
                frame True {
                }
              }
            }
            n99 = Array Size(array=w255) -> (size(s)=w257:i32)
            n100 = for {
              N: w257 -> [_]
              shift-right: [w275] -> w245
              shift-left: w255 -> [w276]
              shift-right: [w273] -> _
              shift-left: 0 -> [w274]
              # "Remove Empty Array"
              n101 = Index Array(array=w276, index=w274) -> (element=w278:string)
              n102 = Equal?(x=w278, y="") -> (x = y?=w277:bool)
              n103 = case shown="True" w277 {
                tunnel: w276 -> [w282 w285]
                tunnel: w274 -> [w281 w283]
                tunnel: [w282 w284] -> w275
                tunnel: [w280 w283] -> w273
                frame False {
                  n104 = Increment(x=w281) -> (x+1=w280:i32)
                }
                frame True {
                  n105 = Delete From Array(array=w285, index=w283) -> (array with subset deleted=w284:string[])  [unwired: 1 in, 1 out]
                }
              }
            }
            "File List" <- w245
            n106 = for {
              tunnel: w245 -> [w271] mode=indexing
              tunnel: [w269] -> w244 mode=indexing
              # "Specify destination path for each file"
              n107 = Concatenate Strings("C:\\temp\\", w271) -> (w270:string)
              n108 = String To Path(string=w270) -> (path=w269:path)
            }
          }
          frame #2 {
            # "FTP a list of files"
            n109 = call <vilib>:"System Exec.vi"("wait until completion? (T)"=TRUE, "working directory"=path "C:/temp", "standard input"=w298, "command line"="C:\\temp\\transfer_ascii_files.bat") -> ()  [unwired: 4 in, 4 out]
          }
          frame #3 {
            # "Move file from local PC to Flight Folder"
            n110 = Build Path(base path=path "\\\\192.168.101.180\\flt_folders" ("path"), name or relative path=w303) -> (appended path=w310:path)
            n111 = Concatenate Strings(w303, "_" ("string"), "corechem" ("string")) -> (w309:string)
            n112 = Build Path(base path=w310, name or relative path=w309) -> (appended path=w305:path)
            n113 = Create Folder(path (use dialog)=w305) -> (created path=w304:path, error out=→"Create folder error out 2":errorcluster)  [unwired: 2 in, 1 out]
            n114 = for {
              tunnel: w304 -> [w317]
              tunnel: [w316] -> w307
              tunnel: w308 -> [w314] mode=indexing
              n115 = Copy(9:TRUE ("overwrite (F)"), 10:w317, 11:w314) -> (0:w316:errorcluster)  [unwired: 2 in, 2 out]
            }
            "Move to FM Error out" <- w307
          }
          frame #4 {
            n116 = local write "FTP ASCII Files to Local"(FALSE ("FTP Files to Local")) -> ()
          }
        }
      }
      event "Transfer FGGA Files": Value Change {
        n117 = event-data() -> ()  [unwired: 1 in, 6 out]
        n118 = flat-sequence {
          tunnel: [w323] -> w322
          tunnel: w322 -> [w335]
          tunnel: [w335] -> w321
          tunnel: [w334] -> w320
          tunnel: [w333] -> w319
          tunnel: w321 -> [w345]
          tunnel: w320 -> [w344]
          tunnel: w319 -> [w346]
          frame #0 {
            n119 = local read "Flight Number"() -> (w324:string)
            n120 = Concatenate Strings("Confirm Flight Number" ("message"), "\n", w324) -> (w326:string)
            n121 = Two Button Dialog(message=w326, 1:"No" ("F button name (\"Cancel\")"), 2:"Yes" ("T button name (\"OK\")")) -> (T button?=w330:bool)
            n122 = case shown="False" w330 {
              tunnel: w324 -> [_ w332]
              tunnel: [w331 w332] -> w323
              frame False {
                n123 = call "Prompt User for Flight Number"() -> ("Flight Number BXXX"=w331:string)  [unwired: 17 in, 2 out]
              }
              frame True {
              }
            }
          }
          frame #1 {
            n124 = Two Button Dialog(message="Get FGGA Files\nof Today's Date?", 1:"No" ("F button name (\"Cancel\")"), 2:"Yes" ("T button name (\"OK\")")) -> (T button?=w339:bool)
            n125 = case shown="False" w339 {
              selector: w339 -> [w341 w342]
              tunnel: [w341 w342] -> w333
              tunnel: [w340 _] -> w334
              frame False {
                n126 = call "Prompt User for Date"() -> ("Date"=w340:string)  [unwired: 17 in, 2 out]
              }
              frame True {
              }
            }
          }
          frame #2 {
            n127 = Build Path(base path=path "\\\\192.168.101.180\\flt_folders" ("path"), name or relative path=w345) -> (appended path=w350:path)
            n128 = Concatenate Strings(w345, "_" ("string"), "corechem" ("string")) -> (w349:string)
            n129 = Build Path(base path=w350, name or relative path=w349) -> (appended path=w343:path)
            n130 = Create Folder(path (use dialog)=w343) -> (error out=→"Create folder error out":errorcluster)  [unwired: 2 in, 2 out]
            n131 = call "labSSH_FGGA_Files_Transfer.vi"("Flight_num"=w345, "Get current?"=w346, "Date"=w344, "Flight Folder Path"=w343) -> ("error IO"=→"FGGA File Transfer Error out":errorcluster)  [unwired: 11 in]
          }
          frame #3 {
            n132 = local write "Transfer FGGA Files"(FALSE) -> ()
          }
        }
      }
      event "FGGA Restart": Value Change {
        n133 = event-data() -> ()  [unwired: 1 in, 6 out]
        n134 = flat-sequence {
          frame #0 {
            n135 = Two Button Dialog(message="FGGA will be restarted,\nARE YOU SURE?") -> (T button?=w356:bool)  [unwired: 2 in]
            n136 = case shown="True" w356 {
              frame False {
              }
              frame True {
                n137 = call "labSSH_Commands.vi"("Data"="reboot") -> ()  [unwired: 14 in, 1 out]
              }
            }
          }
          frame #1 {
            n138 = local write "FGGA Restart"(FALSE ("FGGA Restart")) -> ()
          }
        }
      }
      event "FGGA Shutdown": Value Change {
        n139 = event-data() -> ()  [unwired: 1 in, 6 out]
        n140 = flat-sequence {
          frame #0 {
            n141 = Two Button Dialog(message="FGGA will be shutdown,\nARE YOU SURE?") -> (T button?=w360:bool)  [unwired: 2 in]
            n142 = case shown="True" w360 {
              frame False {
              }
              frame True {
                n143 = call "labSSH_Commands.vi"("Data"="halt") -> ()  [unwired: 14 in, 1 out]
              }
            }
          }
          frame #1 {
            n144 = local write "FGGA Shutdown"(FALSE ("FGGA Restart")) -> ()
          }
        }
      }
    }
    n145 = node-c288() -> ()  [unwired: 1 in, 1 out]
  }
  n146 = while {
    shift-right: [w459] -> _
    shift-left: w8 -> [w457]
    shift-right: [w461] -> _
    shift-left: w7 -> [w462]
    shift-right: [w460] -> _
    shift-left: w9 -> [w464]
    shift-right: [w453] -> _
    shift-left: w9 -> [w455]
    shift-right: [w450] -> _
    shift-left: w8 -> [w449]
    shift-right: [w452] -> _
    shift-left: w7 -> [w454]
    shift-right: [w446] -> _
    shift-left: FALSE -> [w447]
    stop <- FALSE stop-if-true
    w393 = ""
    w388 = "%s" ("format string")
    w583 = "%s" ("format string")
    w588 = "%s" ("format string")
    w593 = "%s" ("format string")
    w599 = "%s" ("format string")
    w605 = "%s" ("format string")
    w609 = "%s" ("format string")
    # "UDP Data Processing"
    n147 = local read "CHFGGA01"() -> (w612:string)
    n148 = local read "TWBOZO01"() -> (w587:string)
    n149 = local read "AL52CO01"() -> (w604:string)
    n150 = local read "CABOZO01"() -> (w592:string)
    n151 = local read "TEIOZO01"() -> (w598:string)
    n152 = local read "CHTSOO01"() -> (w582:string)
    n153 = local read "PRTAFT_UDP_In"() -> (w386:string)
    n154 = local read "Ambient = OFF\nCabin = ON"() -> (w486:bool)
    n155 = Spreadsheet String To Array(delimiter (Tab)=",", format string=w609, spreadsheet string=w612, array type (2D Dbl)=string[] []) -> (array=w559:string[])
    n156 = Spreadsheet String To Array(delimiter (Tab)=",", format string=w605, spreadsheet string=w604, array type (2D Dbl)=string[] []) -> (array=w580:string[])
    n157 = Spreadsheet String To Array(delimiter (Tab)=",", format string=w593, spreadsheet string=w592, array type (2D Dbl)=string[] []) -> (array=w483:string[])
    n158 = Spreadsheet String To Array(delimiter (Tab)=",", format string=w599, spreadsheet string=w598, array type (2D Dbl)=string[] []) -> (array=w557:string[])
    n159 = Spreadsheet String To Array(delimiter (Tab)=",", format string=w588, spreadsheet string=w587, array type (2D Dbl)=string[] []) -> (array=w482:string[])
    n160 = Spreadsheet String To Array(delimiter (Tab)=",", format string=w583, spreadsheet string=w582, array type (2D Dbl)=string[] []) -> (array=w555:string[])
    n161 = Array To Spreadsheet String(delimiter (Tab)="\r", array=w559, 3:w609) -> (spreadsheet string=→"FGGA":string)
    n162 = Array To Spreadsheet String(delimiter (Tab)="\r", array=w580, 3:w605) -> (spreadsheet string=→"CO":string)
    n163 = Array To Spreadsheet String(delimiter (Tab)="\r", array=w483, 3:w593) -> (spreadsheet string=→"Cabin Ozone":string)
    n164 = Array To Spreadsheet String(delimiter (Tab)="\r", array=w557, 3:w599) -> (spreadsheet string=→"Ozone":string)
    n165 = Spreadsheet String To Array(delimiter (Tab)=",", format string=w388, spreadsheet string=w386, array type (2D Dbl)=string[] []) -> (array=w387:string[])
    n166 = Array To Spreadsheet String(delimiter (Tab)="\r", array=w482, 3:w588) -> (spreadsheet string=→"Ambient Ozone":string)
    n167 = Array To Spreadsheet String(delimiter (Tab)="\r", array=w555, 3:w583) -> (spreadsheet string=→"SO2":string)
    n168 = Array To Spreadsheet String(delimiter (Tab)="\r", array=w387, 3:w388) -> (spreadsheet string=→"PRTAFT_DLU":string)
    n169 = Index Array(array=w387, index #1=5 ("index"), index #2=19 ("index")) -> (element #1=w391:string, element #2=w389:string)
    n170 = Select(t=w483, s=w486, f=w482) -> (s? t:f=w481:string[])
    n171 = Not Equal?(x=w391, y=w393) -> (x != y?=w392:bool)
    n172 = Not Equal?(x=w389, y=w393) -> (x != y?=w390:bool)
    n173 = Index Array(array=w555, index #1=6 ("index"), index #2=4 ("index"), index #3=3 ("index"), index #4=7 ("index"), index #5=8 ("index"), index #6=15 ("index"), index #7=24 ("index"), index #8=29 ("index")) -> (element #1=w472:string, element #2=w538:string, element #3=w533:string, element #4=w526:string, element #5=w502:string, element #6=w501:string, element #7=w411:string, element #8=w410:string)
    n174 = Index Array(array=w481, index #1=8 ("index"), index #2=11 ("index")) -> (element #1=w475:string, element #2=w476:string)
    n175 = Index Array(array=w557, index #1=6 ("index"), index #2=4 ("index"), index #3=3 ("index"), index #4=7 ("index"), index #5=9 ("index"), index #6=14 ("index"), index #7=15 ("index")) -> (element #1=w551:string, element #2=w539:string, element #3=w534:string, element #4=w519:string, element #5=w492:string, element #6=w491:string, element #7=w490:string)
    n176 = case shown="False" w390 {
      tunnel: ["1" w618] -> w383
      tunnel: w389 -> [_ w618]
      frame False {
      }
      frame True {
      }
    }
    n177 = case shown="False" w392 {
      tunnel: ["XXXX" w620] -> w384
      tunnel: w391 -> [_ w620]
      frame False {
      }
      frame True {
      }
    }
    n178 = Scan Value(string=w475, format string="%f") -> (value=→"2B Ozone concentration":dbl)  [unwired: 1 in, 1 out]
    n179 = Scan Value(string=w476, format string="%f") -> (value=→"2B Ozone flow rate":dbl)  [unwired: 1 in, 1 out]
    n180 = Scan Value(string=w411, format string="%f") -> (value=→"TEI43i MFC2 Cal Flow":dbl)  [unwired: 1 in, 1 out]
    n181 = Scan Value(string=w410, format string="%f") -> (value=→"TEI43i MFC3 Sample Flow":dbl)  [unwired: 1 in, 1 out]
    n182 = Scan Value(string=w502, format string="%f") -> (value=→"TEi43C / TEi43i Concentration":dbl)  [unwired: 1 in, 1 out]
    n183 = Scan Value(string=w501, format string="%f") -> (value=→"TEI43C Sample Flow":dbl)  [unwired: 1 in, 1 out]
    n184 = Index Array(array=w559, index #1=6 ("index"), index #2=4 ("index"), index #3=3 ("index"), index #4=7 ("index"), index #5=8 ("index"), index #6=9 ("index"), index #7=10 ("index"), index #8=17 ("index"), index #9=16 ("index"), index #10=11 ("index"), index #11=12 ("index"), index #12=21 ("index"), index #13=14 ("index"), index #14=15 ("index")) -> (element #1=w553:string, element #2=w541:string, element #3=w536:string, element #4=w521:string, element #5=w435:string, element #6=w432:string, element #7=w427:string, element #8=w425:string, element #9=w422:string, element #10=w417:string, element #11=w416:string, element #12=w403:string, element #13=w367:string, element #14=w366:string)
    n185 = local write "WoW Flag"(w383) -> ()
    n186 = local write "Flight Number"(w384) -> ()
    n187 = Index Array(array=w580, index #1=2 ("index"), index #2=27 ("index"), index #3=28 ("index"), index #4=29 ("index"), index #5=30 ("index"), index #6=31 ("index"), index #7=6 ("index"), index #8=4 ("index"), index #9=3 ("index"), index #10=8 ("index"), index #11=14 ("index"), index #12=16 ("index"), index #13=19 ("index"), index #14=12 ("index"), index #15=13 ("index"), index #16=10 ("index"), index #17=11 ("index"), index #18=15 ("index")) -> (element #1=w445:string, element #2=w523:string, element #3=w570:string, element #4=w564:string, element #5=w562:string, element #6=w563:string, element #7=w552:string, element #8=w540:string, element #9=w535:string, element #10=w524:string, element #11=w511:string, element #12=w508:string, element #13=w507:string, element #14=w467:string, element #15=w466:string, element #16=w399:string, element #17=w380:string, element #18=w374:string)